vi "UHR-Fleezers Control (host) - 10.5.vi"() -> ()   [LabVIEW 2010] (continued)
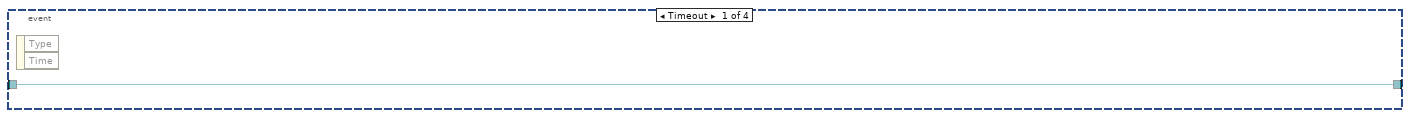
[diagram p2: hidden frame]
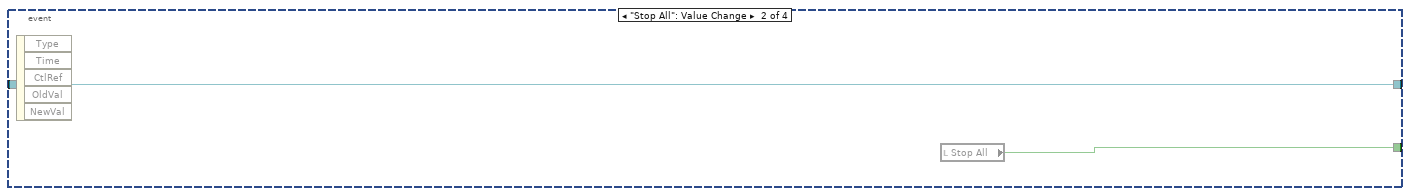
[diagram p3: hidden frame]
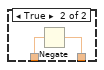
[diagram p4: hidden frame]
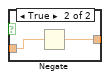
[diagram p5: hidden frame]
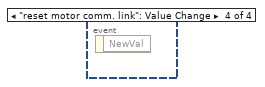
[diagram p6: hidden frame]
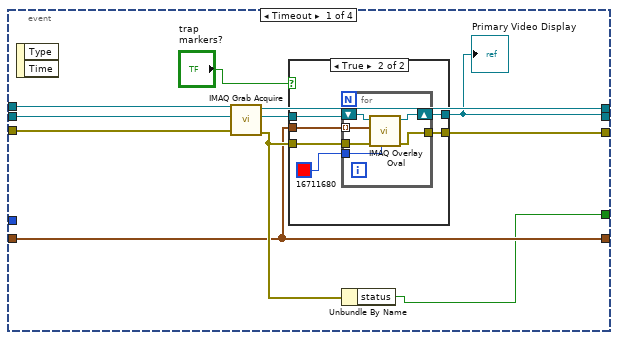
[diagram p8: hidden frame]
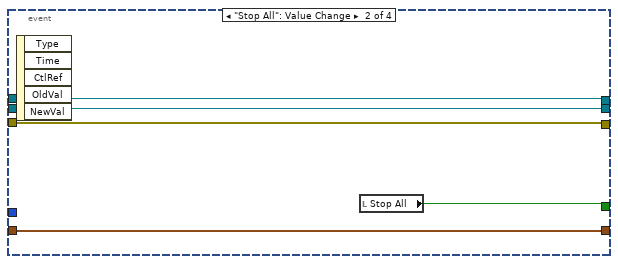
[diagram p10: hidden frame]
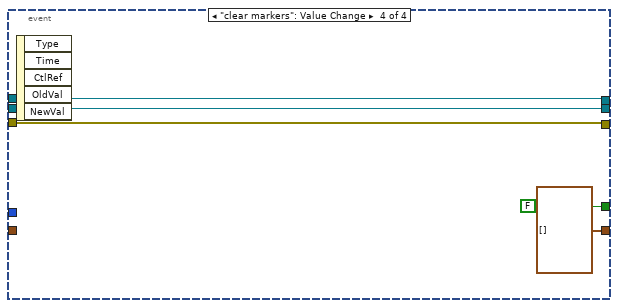
[diagram p12: hidden frame]
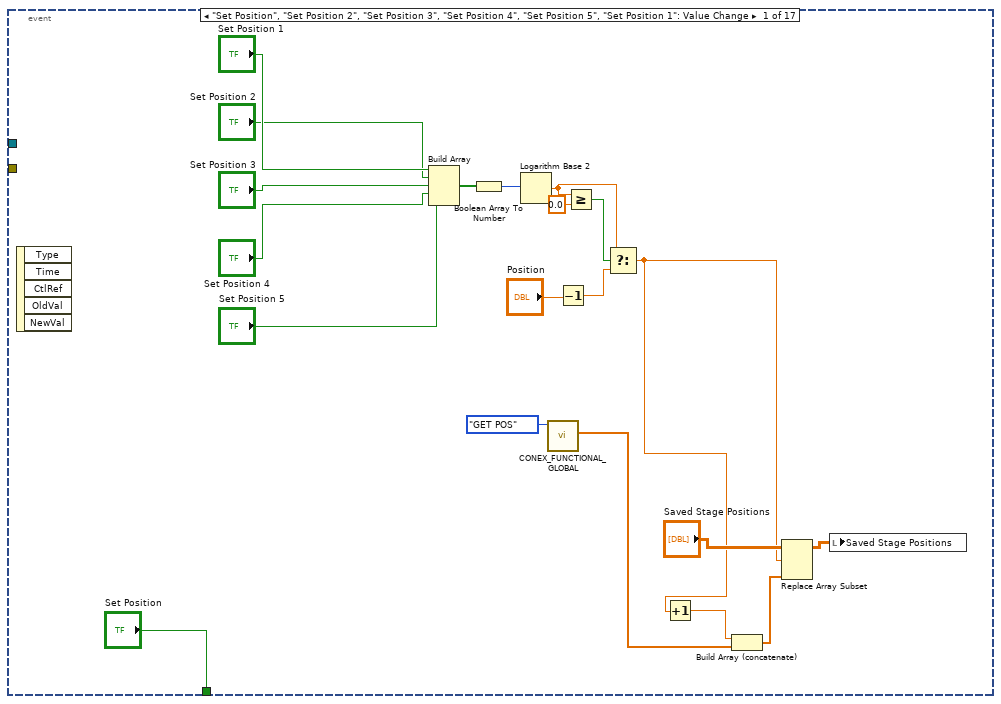
[diagram p13: hidden frame]
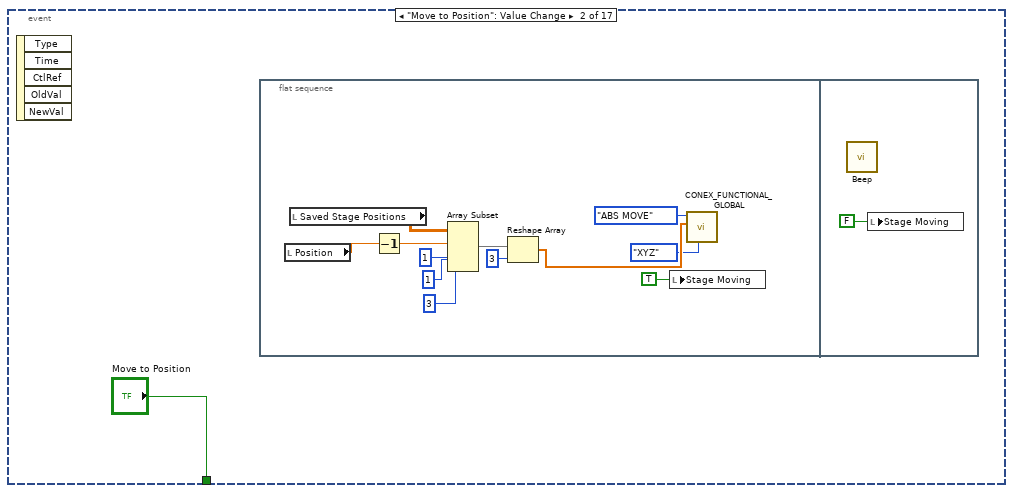
[diagram p14: hidden frame]
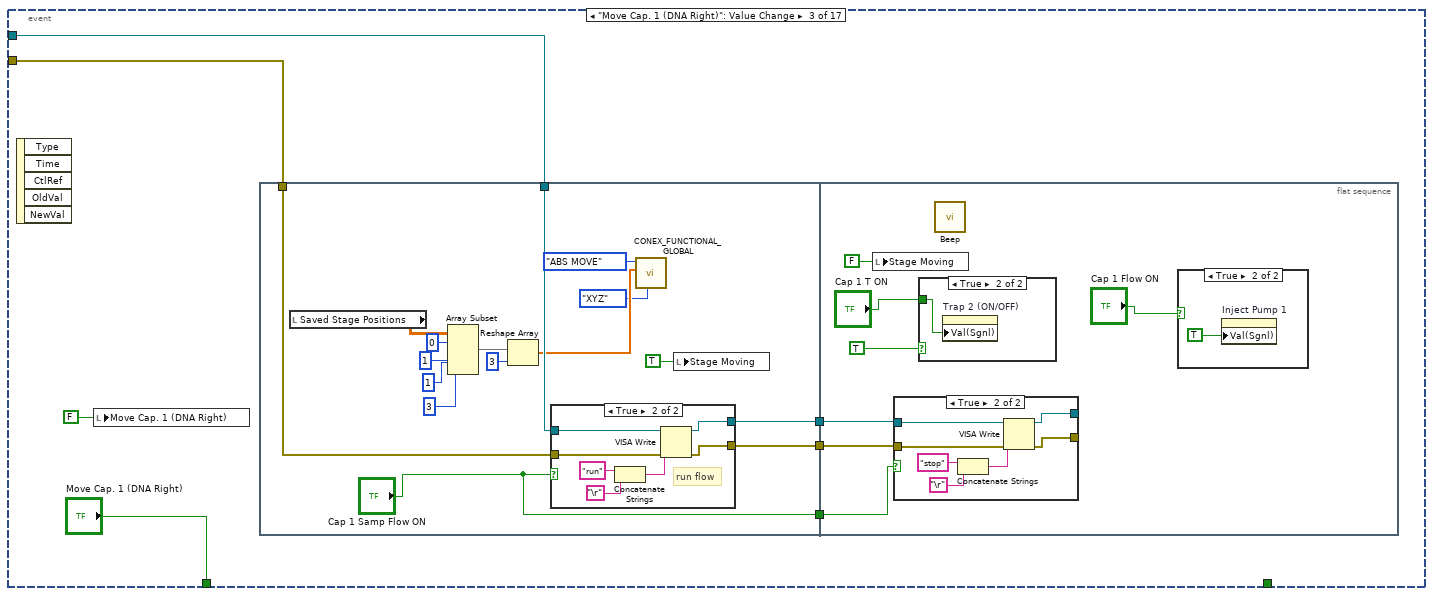
[diagram p15: hidden frame]
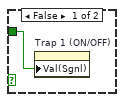
[diagram p19: hidden frame]
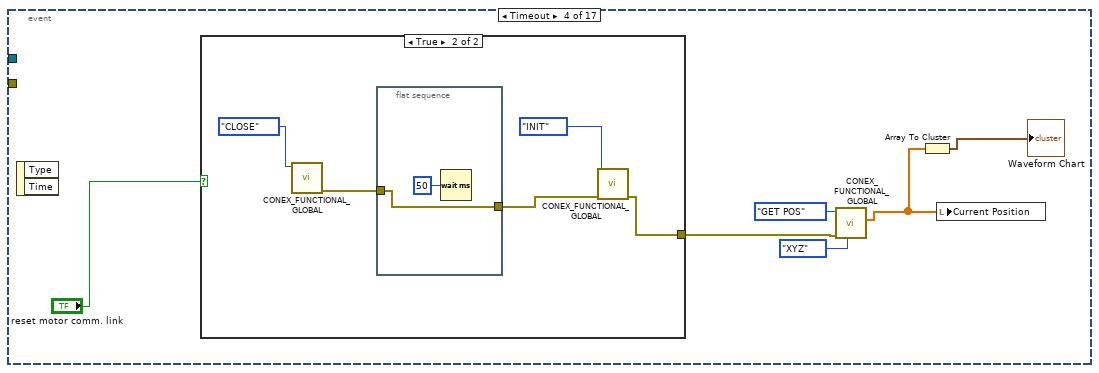
[diagram p20: hidden frame]
            n1941 = property on="Green laser mode" class="RadioBtnsControl (strict)"("Val(Sgnl)"=enum32{"Laser ON", "Laser OFF", "Interlace"}."Laser ON" ("Value (Signaling)")) -> ()  [unwired: 2 in, 2 out]
          }
          frame #3 {
            n1942 = Wait (ms)(milliseconds to wait=u32 500) -> ()  [unwired: 1 out]
          }
          frame #4 {
            n1943 = property on="Confocal Image" class="Bool (strict)"("Val(Sgnl)"=TRUE ("Value (Signaling)")) -> ()  [unwired: 2 in, 2 out]
          }
          frame #5 {
            n1944 = Wait (ms)(milliseconds to wait=u32 2000) -> ()  [unwired: 1 out]
          }
          frame #6 {
            n1945 = while {
              stop <- w8337 stop-if-true
              n1946 = local read "Saving..."() -> (w8338:bool)
              n1947 = Not(x=w8338) -> (.not. x?=w8337:bool)
            }
          }
          frame #7 {
            n1948 = property on="Flip Green Filter" class="Bool (strict)"("Val(Sgnl)"=TRUE ("Value (Signaling)")) -> ()  [unwired: 2 in, 2 out]
            n1949 = property on="Green Laser ON/Interlacing" class="Bool (strict)"("Val(Sgnl)"=w8342) -> ()  [unwired: 2 in, 2 out]
            n1950 = property on="Green laser mode" class="RadioBtnsControl (strict)"("Val(Sgnl)"=w8341) -> ()  [unwired: 2 in, 2 out]
          }
          frame #8 {
            n1951 = property on="Green FB On/Off" class="Bool (strict)"("Val(Sgnl)"=w8343) -> ()  [unwired: 2 in, 2 out]
          }
        }
      }
      event "Stop All": Value Change {
        n1952 = event-data() -> ()  [unwired: 1 in, 5 out]
        n1953 = local read "Stop All"() -> (w8344:bool)
      }
    }
    n1954 = node-c288() -> ()  [unwired: 1 in, 1 out]
  }
  n1955 = timed-loop "Mouse control: trap position (AOM deflection), set confocal spot from image" {
    tunnel: [w8346] -> w12
    tunnel: w9 -> [w8345]
    timing: w81 -> [_]
    timing-out: [_] -> w80
    stop <- w8346 stop-if-true
    n1956 = node-c288() -> ()  [unwired: 2 out]
    n1957 = event shown="[1] \"Pane\": Mouse Move" {
      selector: _ -> [_ _]
      dyn-events: _ -> [_ _]
      timeout: _ -> [_ _]
      tunnel: w8345 -> [w8349 _]
      event Mouse Down {
        n1958 = event-data() -> ("Time"=w8351:u32, "Coords"=w8350:T8, "Button"=w8352:u16)  [unwired: 6 out]
        n1959 = case shown="1" w8352 {
          tunnel: w8351 -> [_ _ w8455]
          tunnel: w8350 -> [_ w8389 w8453]
          tunnel: w8349 -> [_ _ w8451]
          frame 0, Default {
          }
          frame 1 {
            n1960 = property on="APD 2" class="ImageControl"() -> ("Displayed Image Position"=w8359:cluster{"Left":i32, "Top":i32})  [unwired: 2 in, 2 out]
            n1961 = property on="APD 1" class="ImageControl"() -> ("Displayed Image Position"=w8388:cluster{"Left":i32, "Top":i32})  [unwired: 2 in, 2 out]
            n1962 = property on="Detection Laser X" class="ImageControl"() -> ("Displayed Image Position"=w8385:cluster{"Left":i32, "Top":i32})  [unwired: 2 in, 2 out]
            n1963 = property on="Detection Laser Y" class="ImageControl"() -> ("Displayed Image Position"=w8384:cluster{"Left":i32, "Top":i32})  [unwired: 2 in, 2 out]
            n1964 = property on="APD 2" class="ImageControl"() -> ("Displayed Image Size"=w8358:cluster{"Width":u32, "Height":u32})  [unwired: 2 in, 2 out]
            n1965 = property on="APD 1" class="ImageControl"() -> ("Displayed Image Size"=w8386:cluster{"Width":u32, "Height":u32})  [unwired: 2 in, 2 out]
            n1966 = property on="Detection Laser X" class="ImageControl"() -> ("Displayed Image Size"=w8387:cluster{"Width":u32, "Height":u32})  [unwired: 2 in, 2 out]
            n1967 = property on="Detection Laser Y" class="ImageControl"() -> ("Displayed Image Size"=w8383:cluster{"Width":u32, "Height":u32})  [unwired: 2 in, 2 out]
            n1968 = Unbundle By Name(w8358) -> ("Width"=w8355:u32, "Height"=w8354:u32)
            n1969 = Unbundle By Name(w8359) -> ("Left"=w8357:i32, "Top"=w8356:i32)
            n1970 = Unbundle By Name(w8386) -> ("Width"=w8380:u32, "Height"=w8379:u32)
            n1971 = Unbundle By Name(w8387) -> ("Width"=w8376:u32, "Height"=w8375:u32)
            n1972 = Unbundle By Name(w8383) -> ("Width"=w8372:u32, "Height"=w8371:u32)
            n1973 = Unbundle By Name(w8388) -> ("Left"=w8382:i32, "Top"=w8381:i32)
            n1974 = Unbundle By Name(w8385) -> ("Left"=w8378:i32, "Top"=w8377:i32)
            n1975 = Unbundle By Name(w8384) -> ("Left"=w8374:i32, "Top"=w8373:i32)
            n1976 = Bundle("Left"=w8357, "Top"=w8356, "Width"=w8355, "Height"=w8354) -> (w8353:T50)  [unwired: 1 in]
            n1977 = Bundle("Left"=w8382, "Top"=w8381, "Width"=w8380, "Height"=w8379) -> (w8370:T50)  [unwired: 1 in]
            n1978 = Bundle("Left"=w8378, "Top"=w8377, "Width"=w8376, "Height"=w8375) -> (w8369:T50)  [unwired: 1 in]
            n1979 = Bundle("Left"=w8374, "Top"=w8373, "Width"=w8372, "Height"=w8371) -> (w8368:T50)  [unwired: 1 in]
            n1980 = Build Cluster Array(w8353, w8370, w8369, w8368) -> (w8367:T51)
            n1981 = for {
              tunnel: w8389 -> [w8400]
              tunnel: w8367 -> [w8401] mode=indexing
              shift-right: [w8398] -> w8365
              shift-left: TRUE -> [w8399]
              shift-right: [w8397] -> w8363
              shift-left: _ -> [w8393]
              shift-right: [w8396] -> w8362
              shift-left: _ -> [w8392]
              shift-right: [w8395] -> w8361
              shift-left: _ -> [w8391]
              shift-right: [w8394] -> w8360
              shift-left: _ -> [w8390]
              n1982 = case shown="True" w8399 {
                selector: w8399 -> [w8406 _]
                tunnel: w8401 -> [_ w8415]
                tunnel: w8400 -> [_ w8413]
                tunnel: [w8406 w8411] -> w8398
                tunnel: [w8405 w8410] -> w8397
                tunnel: [w8404 w8409] -> w8396
                tunnel: [w8403 w8408] -> w8395
                tunnel: [w8402 w8407] -> w8394
                tunnel: w8393 -> [w8405 _]
                tunnel: w8392 -> [w8404 _]
                tunnel: w8391 -> [w8403 _]
                tunnel: w8390 -> [w8402 _]
                frame False {
                }
                frame True {
                  n1983 = Unbundle(w8415) -> (w8414:T50)
                  n1984 = call "isclickinwindow.vi"("Image Param"=w8414, "Point32"=w8413) -> ("4 Y"=w8407:i32, "3 Height"=w8408:i32, "2 X"=w8409:i32, "1 Width"=w8410:i32, "In image?"=w8412:bool)  [unwired: 1 in]
                  n1985 = Not(x=w8412) -> (.not. x?=w8411:bool)
                }
              }
            }
            n1986 = Not(x=w8365) -> (.not. x?=w8364:bool)
            n1987 = case shown="True" w8364 {
              tunnel: w8362 -> [_ w8428]
              tunnel: w8360 -> [_ w8427]
              tunnel: w8363 -> [_ w8426]
              tunnel: w8361 -> [_ w8425]
              frame False {
              }
              frame True {
                w8421 = FALSE ("Get Point")
                n1988 = local read "Scan lines (y)"() -> (w8430:u64)
                n1989 = local read "Actual MCL Inc (V)"() -> (w8422:dbl)
                n1990 = local read "Scan steps (MCL)"() -> (w8429:u64)
                n1991 = Divide "Y Pix/step"(x=w8425, y=w8430) -> (x/y=w8437:dbl)
                n1992 = Divide "Y V/pix"(x=w8422, y=w8437) -> (x/y=w8436:dbl)
                n1993 = Divide "Y half step offset"(x=w8422, y=2.0) -> (x/y=w8438:dbl)
                n1994 = Divide "X pix/step"(x=w8426, y=w8429) -> (x/y=w8435:dbl)
                n1995 = Negate(x=w8438) -> (-x=w8439:dbl)
                n1996 = local read "Initial Y"() -> (w8445:dbl)
                n1997 = Multiply(x=w8427, y=w8436) -> (x*y=w8446:dbl)
                n1998 = Divide "X half step offset"(x=w8422, y=2.0) -> (x/y=w8432:dbl)
                n1999 = Divide "X V/pix"(x=w8422, y=w8435) -> (x/y=w8434:dbl)
                n2000 = Multiply(x=w8422, y=w8429) -> (x*y=w8441:dbl)
                n2001 = Compound Arithmetic op=ADD(w8439, w8446, w8445) -> (w8423:dbl)
                "Pointer Y (V)" <- w8423
                n2002 = Multiply(x=w8434, y=w8428) -> (x*y=w8443:dbl)
                n2003 = Negate(x=w8432) -> (-x=w8431:dbl)
                n2004 = local read "Initial X"() -> (w8444:dbl)
                n2005 = Negate(x=w8443) -> (-x=w8442:dbl)
                n2006 = Compound Arithmetic op=ADD(w8431, w8441, w8444, w8442) -> (w8424:dbl)
                "Pointer X (V)" <- w8424
                n2007 = Or(x="Set X Only", y="Set Confocal Spot (X-Y)") -> (x .or. y?=w8417:bool)
                n2008 = Or(x="Set Confocal Spot (X-Y)", y="Set Y Only") -> (x .or. y?=w8416:bool)
                n2009 = case shown="True" w8417 {
                  tunnel: w8424 -> [_ w8447]
                  frame False {
                  }
                  frame True {
                    n2010 = property on="AO2" class="Slide (strict)"("Val(Sgnl)"=w8447) -> ()  [unwired: 2 in, 2 out]
                  }
                }
                n2011 = case shown="True" w8416 {
                  tunnel: w8423 -> [_ w8448]
                  frame False {
                  }
                  frame True {
                    n2012 = property on="AO1" class="Slide (strict)"("Val(Sgnl)"=w8448) -> ()  [unwired: 2 in, 2 out]
                  }
                }
                n2013 = local write "Set Confocal Spot (X-Y)"(w8421) -> ()
                n2014 = local write "Set X Only"(w8421) -> ()
                n2015 = local write "Set Y Only"(w8421) -> ()
              }
            }
          }
          frame 3 {
            n2016 = local read "BD 2 Frequency 1 (MHz)"() -> (w8449:dbl)
            n2017 = local read "BD 1 Frequency 1 (MHz)"() -> (w8450:dbl)
            n2018 = local write "Manipulating Trap"(TRUE ("Manipulating Trap")) -> ()
            n2019 = local write "Coords"(T8 {"Horizontal"=0, "Vertical"=0} ("Coords")) -> ()
            n2020 = while {
              tunnel: w8455 -> [w8460]
              tunnel: w8453 -> [w8459]
              tunnel: w8451 -> [w8458]
              tunnel: w8450 -> [w8457]
              tunnel: w8449 -> [w8456]
              stop <- w8461 stop-if-true
              n2021 = event shown="[0] \"Pane\": Mouse Move" {
                selector: _ -> [_ _]
                dyn-events: _ -> [_ _]
                timeout: _ -> [_ _]
                tunnel: ["Force Manip Abort" w8525] -> w8461
                tunnel: w8460 -> [w8468 _]
                tunnel: w8459 -> [w8466 _]
                tunnel: w8458 -> [w8465 _]
                tunnel: w8457 -> [w8464 _]
                tunnel: w8456 -> [w8463 _]
                event Mouse Move {
                  n2022 = event-data() -> ("Time"=w8469:u32, "Coords"=w8470:T8)  [unwired: 3 out]
                  n2023 = Less?(x=w8469, y=w8468) -> (x < y?=w8467:bool)
                  n2024 = case "Makes sure old motion events prior to mouse click aren't used" shown="False" w8467 {
                    tunnel: w8470 -> [w8512 _]
                    tunnel: w8466 -> [w8513 _]
                    tunnel: w8465 -> [w8490 _]
                    tunnel: w8464 -> [w8486 _]
                    tunnel: w8463 -> [w8485 _]
                    frame False {
                      n2025 = Subtract(x=w8512, y=w8513) -> (x-y=w8511:T8)
                      "Coords" <- w8511
                      n2026 = local read "Y RF Frequency Limits (MHz)"() -> (w8471:T17)
                      n2027 = To Double Precision Float(number=w8511) -> (double precision float=w8510:cluster{"Horizontal":dbl, "Vertical":dbl})
                      n2028 = Multiply(x=cluster{"Horizontal":dbl, "Vertical":dbl} {"Horizontal"=-1.0, "Vertical"=1.0}, y="Manipulation Scaling") -> (x*y=w8506:cluster{"Horizontal":dbl, "Vertical":dbl})
                      n2029 = local read "X RF Frequency Limits (MHz)"() -> (w8472:T17)
                      n2030 = Multiply(x=w8510, y=w8506) -> (x*y=w8508:cluster{"Horizontal":dbl, "Vertical":dbl})
                      n2031 = Unbundle By Name(w8508) -> ("Horizontal"=w8503:dbl, "Vertical"=w8507:dbl)
                      n2032 = Unbundle By Name(w8471) -> ("Maximum"=w8474:dbl, "Minimum"=w8473:dbl)
                      n2033 = Boolean To (0,1)(Boolean="Manip. X?") -> (0, 1=w8501:i16)
                      n2034 = Boolean To (0,1)(Boolean="Manip. Y?") -> (0, 1=w8498:i16)
                      n2035 = local read "BD 1 Frequency 2 (MHz)"() -> (w8488:dbl)
                      n2036 = Multiply(x=w8507, y=w8498) -> (x*y=w8500:dbl)
                      n2037 = Multiply(x=w8501, y=w8503) -> (x*y=w8504:dbl)
                      n2038 = local read "BD 2 Frequency 2 (MHz)"() -> (w8487:dbl)
                      n2039 = Unbundle By Name(w8472) -> ("Maximum"=w8476:dbl, "Minimum"=w8475:dbl)
                      n2040 = Add(x=w8485, y=w8500) -> (x+y=w8478:dbl)
                      n2041 = Add(x=w8486, y=w8504) -> (x+y=w8480:dbl)
                      n2042 = In Range and Coerce(upper limit=w8476, x=w8480, lower limit=w8475) -> (coerced(x)=w8479:dbl)  [unwired: 1 out]
                      n2043 = In Range and Coerce(upper limit=w8474, x=w8478, lower limit=w8473) -> (coerced(x)=w8477:dbl)  [unwired: 1 out]
                      n2044 = Subtract(x=w8479, y=w8488) -> (x-y=w8497:dbl)
                      n2045 = Subtract(x=w8477, y=w8487) -> (x-y=w8496:dbl)
                      n2046 = Square(x=w8497) -> (x^2=w8495:dbl)
                      n2047 = Square(x=w8496) -> (x^2=w8494:dbl)
                      n2048 = Add(x=w8495, y=w8494) -> (x+y=w8493:dbl)
                      n2049 = Square Root(x=w8493) -> (sqrt(x)=w8489:dbl)
                      n2050 = In Range and Coerce(upper limit="Limit Max (MHz)", x=w8489, lower limit="Limit Min (MHz)") -> (In Range?=w8482:bool)  [unwired: 1 out]
                      n2051 = Not(x="Limits Enable") -> (.not. x?=w8481:bool)
                      n2052 = Or(x=w8482, y=w8481) -> (x .or. y?=w8483:bool)
                      n2053 = case shown="True" w8483 {
                        tunnel: w8490 -> [_ w8523]
                        tunnel: w8489 -> [_ w8514]
                        tunnel: w8479 -> [_ w8521]
                        tunnel: w8488 -> [_ w8520]
                        tunnel: w8477 -> [_ w8519]
                        tunnel: w8487 -> [_ w8518]
                        tunnel: w8472 -> [_ w8516]
                        tunnel: w8471 -> [_ w8515]
                        frame False {
                        }
                        frame True {
                          n2054 = local read "BD 1 Frequency 3 (MHz)"() -> (w8522:dbl)
                          n2055 = local read "BD 2 Frequency 3 (MHz)"() -> (w8517:dbl)
                          n2056 = local write "Trap Delta (MHz)"(w8514) -> ()
                          n2057 = property on="Initial delta (MHz)" class="DigNum (strict)"("Val(Sgnl)"=w8514) -> ()  [unwired: 2 in, 2 out]
                          n2058 = call "set RF board frequency - interlace.vi"("Board 2 Frequency Limits"=w8515, "Board 1 Frequency Limits"=w8516, "FPGA VI Reference In"=w8523, "Board 2 Frequency 3 (MHz)"=w8517, "Board 1 Frequency 3 (MHz)"=w8522, "Board 2 Frequency 2 (MHz)"=w8518, "Board 2 Frequency 1 (MHz)"=w8519, "Board 1 Frequency 2 (MHz)"=w8520, "Board 1 Frequency 1  (MHz)"=w8521) -> ()  [unwired: 1 in, 2 out]
                          n2059 = local write "BD 2 Frequency 1 (MHz)"(w8519) -> ()
                          n2060 = local write "BD 1 Frequency 1 (MHz)"(w8521) -> ()
                        }
                      }
                    }
                    frame True {
                    }
                  }
                }
                event Mouse Up {
                  n2061 = event-data() -> ("Button"=w8524:u16)  [unwired: 8 out]
                  n2062 = case shown="3" w8524 {
                    tunnel: [FALSE TRUE] -> w8525
                    frame 0, Default {
                    }
                    frame 3 {
                      n2063 = local write "Manipulating Trap"(FALSE ("Manipulating Trap")) -> ()
                    }
                  }
                }
              }
            }
          }
        }
      }
      event Mouse Move {
        n2064 = event-data() -> ()  [unwired: 6 out]
      }
    }
    n2065 = local read "Stop All"() -> (w8346:bool)
    n2066 = node-c288() -> ()  [unwired: 2 out]
  }
  n2067 = timed-loop "Oscillate AOD (debugging)" {
    tunnel: w9 -> [w8530]
    tunnel: [w8529] -> w14
    timing: w77 -> [_]
    timing-out: [_] -> w76
    stop <- w8529 stop-if-true
    n2068 = node-c288() -> ()  [unwired: 2 out]
    n2069 = event shown="[2] \"Stop All\": Value Change" {
      selector: _ -> [_ _ _]
      dyn-events: _ -> [_ _ _]
      timeout: _ -> [_ _ _]
      tunnel: w8530 -> [w8537 _ _]
      tunnel: [FALSE ("Stop All") _ w8806] -> w8529
      event "Oscillate Set 1", "Fish for Tether": Value Change {
        n2070 = event-data() -> ()  [unwired: 6 out]
        n2071 = local read "Oscillate Set 1"() -> (w8536:bool)
        n2072 = Or(x=w8536, y="Fish for Tether") -> (x .or. y?=w8534:bool)
        n2073 = case shown="True" w8534 {
          tunnel: w8537 -> [_ w8540]
          tunnel: "Fish for Tether" -> [_ w8539]
          frame False {
          }
          frame True {
            n2074 = case shown="False" w8539 {
              frame False {
              }
              frame True {
                n2075 = local write "Scan axis 2"(TRUE) -> ()
                n2076 = local write "Tether"(FALSE ("Tether")) -> ()
              }
            }
            n2077 = node-c288(i64 50 ("Period")) -> (w8542:T25)  [unwired: 3 out]
            n2078 = timed-loop "Oscillate AOD" {
              timing: w8542 -> [_]
              timing-out: [_] -> w8541
              tunnel: w8540 -> [w8552]
              tunnel: w8539 -> [w8551]
              i -> [w8554]
              stop <- w8550 stop-if-true
              n2079 = node-c288() -> (w8553:i64)  [unwired: 1 out]
              n2080 = flat-sequence {
                tunnel: w8554 -> [w8581]
                tunnel: w8553 -> [w8580]
                tunnel: w8552 -> [w8561]
                tunnel: w8551 -> [w8564]
                tunnel: [w8564] -> w8549
                tunnel: [w8563] -> w8548
                tunnel: [w8560] -> w8547
                tunnel: [w8557] -> w8545
                tunnel: w8549 -> [w8617]
                tunnel: w8548 -> [w8615]
                tunnel: w8547 -> [w8614]
                tunnel: [w8613] -> w8546
                tunnel: w8545 -> [w8612]
                tunnel: [w8681] -> w8550
                tunnel: w8546 -> [w8679]
                frame #0 {
                  n2081 = Divide(x=w8580, y=i64 1000) -> (x/y=w8575:dbl)
                  n2082 = Multiply(x=w8575, y=w8581) -> (x*y=w8577:dbl)
                  n2083 = Multiply(x="Osc. freq. (Hz)", y=6.283185307179586) -> (x*y=w8578:dbl)
                  n2084 = Multiply(x=w8578, y=w8577) -> (x*y=w8559:dbl)
                  n2085 = local read "BD 1 Frequency 2 (MHz)"() -> (w8562:dbl)
                  n2086 = local read "BD 1 Frequency 1 (MHz)"() -> (w8555:dbl)
                  n2087 = case shown="False" w8564 {
                    tunnel: w8559 -> [w8587 w8593]
                    tunnel: w8562 -> [_ w8604]
                    tunnel: [w8584 w8599] -> w8565
                    tunnel: [FALSE w8596] -> w8560
                    tunnel: [0.0 w8589] -> w8557
                    tunnel: w8555 -> [_ w8588]
                    frame False {
                      n2088 = Sine(x=w8587) -> (sin(x)=w8585:dbl)
                      n2089 = Multiply(x=w8585, y="Osc. amp. (MHz)") -> (x*y=w8584:dbl)
                    }
                    frame True {
                      n2090 = Cosine(x=w8593) -> (cos(x)=w8607:dbl)
                      n2091 = Subtract(x=w8604, y=w8588) -> (x-y=w8603:dbl)
                      n2092 = Decrement(x=w8607) -> (x-1=w8606:dbl)
                      n2093 = Subtract(x=w8603, y="Closest Delta (MHz)") -> (x-y=w8600:dbl)
                      n2094 = Divide(x=w8606, y=-2.0) -> (x/y=w8601:dbl)
                      n2095 = Multiply(x=w8601, y=w8600) -> (x*y=w8599:dbl)
                      n2096 = local read "Vec Mean of T1 T2"() -> (w8595:dbl[])
                      n2097 = Greater?(x=w8595, y="Stop F (pN)") -> (0:w8597:bool[])
                      n2098 = Or Array Elements(Boolean array=w8597) -> (logical OR=w8596:bool)
                      n2099 = Divide(x=w8593, y=6.283185307179586) -> (x/y=w8592:dbl)
                      n2100 = Round Toward +Infinity(x=w8592) -> (ceil(x): smallest int >= x=w8589:dbl)
                      "Attempts" <- w8589
                      n2101 = Greater?(x=w8589, y="Attempt Limit") -> (0:w8591:bool)
                      n2102 = case shown="True" w8591 {
                        frame False {
                        }
                        frame True {
                          n2103 = local write "Fish for Tether"(FALSE ("Fish for Tether")) -> ()
                          n2104 = call <vilib>:"Beep.vi"() -> ()  [unwired: 3 in, 9 out]
                          n2105 = local read "Messages"() -> (w8609:string)
                          n2106 = call "Update messages.vi"("Message to add"="Tether fishing timeout." ("Messages"), "Old message string"=w8609) -> ("New message string"=→"Messages":string)
                        }
                      }
                    }
                  }
                  n2107 = local read "BD 2 Frequency 1 (MHz)"() -> (w8566:dbl)
                  n2108 = Select(t=w8555, s="Scan axis 2", f=w8566) -> (s? t:f=w8569:dbl)
                  n2109 = Add(x=w8565, y=w8569) -> (x+y=w8563:dbl)
                  n2110 = Select(t=w8563, s="Scan axis 2", f=w8555) -> (s? t:f=w8556:dbl)
                  n2111 = Select(t=w8566, s="Scan axis 2", f=w8563) -> (s? t:f=w8571:dbl)
                  n2112 = local read "Y RF Frequency Limits (MHz)"() -> (w8567:T17)
                  n2113 = local read "X RF Frequency Limits (MHz)"() -> (w8568:T17)
                  n2114 = local read "BD 1 Frequency 3 (MHz)"() -> (w8574:dbl)
                  n2115 = local read "BD 2 Frequency 2 (MHz)"() -> (w8573:dbl)
                  n2116 = local read "BD 2 Frequency 3 (MHz)"() -> (w8572:dbl)
                  n2117 = call "set RF board frequency - interlace.vi"("Board 2 Frequency Limits"=w8567, "Board 1 Frequency Limits"=w8568, "FPGA VI Reference In"=w8561, "Board 2 Frequency 3 (MHz)"=w8572, "Board 1 Frequency 3 (MHz)"=w8574, "Board 2 Frequency 2 (MHz)"=w8573, "Board 2 Frequency 1 (MHz)"=w8571, "Board 1 Frequency 2 (MHz)"=w8562, "Board 1 Frequency 1  (MHz)"=w8556) -> ()  [unwired: 1 in, 2 out]
                }
                frame #1 {
                  n2118 = And(x=w8617, y=w8614) -> (x .and. y?=w8616:bool)
                  n2119 = case "Only if were fishing and now formed tether" shown="False" w8616 {
                    tunnel: w8615 -> [w8619 w8631]
                    tunnel: [w8618 w8630] -> w8613
                    tunnel: w8612 -> [_ w8626]
                    frame False {
                      n2120 = local read "Fish for Tether"() -> (w8618:bool)
                      n2121 = case shown="False" w8618 {
                        tunnel: w8619 -> [_ _]
                        frame False {
                        }
                        frame True {
                        }
                      }
                    }
                    frame True {
                      w8630 = FALSE ("Fish for Tether")
                      n2122 = call <vilib>:"Beep.vi"() -> ()  [unwired: 3 in, 9 out]
                      n2123 = Number To Decimal String(number=w8626, width (-)=i16 1) -> (decimal integer string=w8624:string)
                      n2124 = case shown="\"1\", Default" "Then..." {
                        selector: "Then..." -> [_ w8634]
                        tunnel: w8631 -> [w8633 _]
                        frame "1", Default {
                          n2125 = property on="BD 1 Frequency 1 (MHz)" class="DigNum (strict)"("Val(Sgnl)"=w8633) -> ()  [unwired: 2 in, 2 out]
                        }
                        frame "2", "3", "4", "5", "6" {
                          n2126 = flat-sequence {
                            tunnel: w8634 -> [w8636]
                            frame #0 {
                              n2127 = property on="Trap Delta (MHz)" class="DigNum (strict)"("Val(Sgnl)"="Move to Delta 1 (MHz)") -> ()  [unwired: 2 in, 2 out]
                            }
                            frame #1 {
                              n2128 = case shown="\"5\", \"6\"" w8636 {
                                selector: w8636 -> [w8639 w8649 _]
                                frame "3", "4" {
                                n2129 = flat-sequence {
                                tunnel: w8639 -> [w8640]
                                tunnel: [w8640] -> w8637
                                tunnel: [w8642] -> w8638
                                tunnel: w8637 -> [w8642]
                                tunnel: w8638 -> [w8646]
                                frame #0 {
                                n2130 = property on="Green Laser ON/Interlacing" class="Bool (strict)"("Val(Sgnl)"=TRUE ("Value (Signaling)")) -> ()  [unwired: 2 in, 2 out]
                                }
                                frame #1 {
                                n2131 = Multiply(x="Wait Before Save (s)", y=u32 1000 ("x")) -> (x*y=w8644:u32)
                                n2132 = Wait (ms)(milliseconds to wait=w8644) -> ()  [unwired: 1 out]
                                }
                                frame #2 {
                                n2133 = property on="Start Saving" class="Bool (strict)"("Value"=TRUE ("Start Saving")) -> ()  [unwired: 2 in, 2 out]
                                n2134 = case shown="\"4\"" w8646 {
                                frame Default {
                                }
                                frame "4" {
                                n2135 = property on="Fl. Triggered..." class="Bool (strict)"("Val(Sgnl)"=TRUE ("Value (Signaling)")) -> ()  [unwired: 2 in, 2 out]
                                }
                                }
                                }
                                }
                                }
                                frame "5", "6" {
                                n2136 = stacked-sequence {
                                tunnel: w8649 -> [_ _ _ _ _ _ _ _ w8666 _ _]
                                frame #0 {
                                n2137 = Replace Array Subset(array=u32[] [0] ("Index Values"), new element="Raster Set Upon Tether", index=0) -> (w8650:u32[])
                                n2138 = property on="Saved AOD Raster Scan Parameter Sets" class="Arr (strict)"("Index Values"=w8650) -> ()  [unwired: 2 in, 2 out]
                                }
                                frame #1 {
                                n2139 = Wait (ms)(milliseconds to wait=u32 500) -> ()  [unwired: 1 out]
                                }
                                frame #2 {
                                n2140 = property on="Load parameters" class="Bool (strict)"("Val(Sgnl)"=TRUE ("Value (Signaling)")) -> ()  [unwired: 2 in, 2 out]
                                }
                                frame #3 {
                                n2141 = Wait (ms)(milliseconds to wait=u32 500) -> ()  [unwired: 1 out]
                                }
                                frame #4 {
                                n2142 = property on="Trap Raster Scan" class="Bool (strict)"("Val(Sgnl)"=TRUE ("Value (Signaling)")) -> ()  [unwired: 2 in, 2 out]
                                }
                                frame #5 {
                                n2143 = Wait (ms)(milliseconds to wait=u32 2000) -> ()  [unwired: 1 out]
                                }
                                frame #6 {
                                n2144 = while {
                                stop <- w8661 stop-if-true
                                n2145 = local read "Raster Scanning..."() -> (w8660:bool)
                                n2146 = local read "Saving..."() -> (w8663:bool)
                                n2147 = Wait (ms)(milliseconds to wait=u32 100) -> ()  [unwired: 1 out]
                                n2148 = Not(x=w8663) -> (.not. x?=w8662:bool)
                                n2149 = Not(x=w8660) -> (.not. x?=w8659:bool)
                                n2150 = And(x=w8662, y=w8659) -> (x .and. y?=w8661:bool)
                                }
                                }
                                frame #7 {
                                n2151 = property on="Trap Delta (MHz)" class="DigNum (strict)"("Val(Sgnl)"="Move to Delta 2 (MHz)") -> ()  [unwired: 2 in, 2 out]
                                }
                                frame #8 {
                                n2152 = local read "Tether"() -> (w8667:bool)
                                n2153 = case shown="True" w8667 {
                                tunnel: w8666 -> [_ w8668]
                                frame False {
                                }
                                frame True {
                                n2154 = flat-sequence {
                                tunnel: w8668 -> [w8670]
                                frame #0 {
                                n2155 = Wait (ms)(milliseconds to wait=u32 500) -> ()  [unwired: 1 out]
                                }
                                frame #1 {
                                n2156 = case shown="\"6\"" w8670 {
                                frame Default {
                                }
                                frame "6" {
                                n2157 = property on="Green Laser ON/Interlacing" class="Bool (strict)"("Val(Sgnl)"=TRUE ("Green Laser ON/Interlacing")) -> ()  [unwired: 2 in, 2 out]
                                }
                                }
                                }
                                frame #2 {
                                n2158 = Wait (ms)(milliseconds to wait=u32 500) -> ()  [unwired: 1 out]
                                }
                                frame #3 {
                                n2159 = local write "Start Saving"("Save at end (5, 6)") -> ()
                                }
                                }
                                }
                                }
                                }
                                frame #9 {
                                n2160 = local read "Bead Sep. Int. Time (s)"() -> (w8676:dbl)
                                n2161 = Multiply(x=w8676, y=1000.0) -> (x*y=w8675:dbl)
                                n2162 = Wait (ms)(milliseconds to wait=w8675) -> ()  [unwired: 1 out]
                                }
                                frame #10 {
                                n2163 = property on="Rescale on Mean" class="Bool (strict)"("Val(Sgnl)"=TRUE ("Value (Signaling)")) -> ()  [unwired: 2 in, 2 out]
                                }
                                }
                                }
                                frame "2", Default {
                                }
                              }
                            }
                          }
                        }
                      }
                      n2164 = Concatenate Strings("Formed tether in ", w8624, " attempt(s)." ("string")) -> (w8621:string)
                      n2165 = local read "Messages"() -> (w8628:string)
                      n2166 = local write "Fish for Tether"(w8630) -> ()
                      n2167 = call "Update messages.vi"("Message to add"=w8621, "Old message string"=w8628) -> ("New message string"=w8627:string)
                      n2168 = local write "Messages"(w8627) -> ()
                      n2169 = Get Date/Time In Seconds() -> (seconds since 1Jan1904=→"Time tether formed":timestamp)
                      "Tether" <- "Tether Alarm?"
                    }
                  }
                }
                frame #2 {
                  n2170 = local read "Oscillate Set 1"() -> (w8680:bool)
                  n2171 = local read "Stop All"() -> (w8682:bool)
                  n2172 = Not Or(1:w8679, 2:w8680) -> (0:w8678:bool)
                  n2173 = Compound Arithmetic op=OR(w8682, w8678) -> (w8681:bool)
                }
              }
              n2174 = node-c288() -> ()  [unwired: 2 out]
            }
            n2175 = node-c288(w8541) -> ()  [unwired: 1 out]
          }
        }
      }
      event "Fl. Triggered...": Value Change {
        n2176 = event-data() -> ()  [unwired: 7 out]
        n2177 = case shown="True" "Fl. Triggered..." {
          frame False {
          }
          frame True {
            n2178 = node-c288() -> (w8694:T25)  [unwired: 4 out]
            n2179 = timed-loop {
              timing: w8694 -> [_]
              timing-out: [_] -> w8693
              tunnel: "Action" -> [w8698]
              shift-right: [w8695] -> _
              shift-left: u8 255 -> [w8697]
              stop <- w8699 stop-if-true
              n2180 = node-c288() -> ()  [unwired: 2 out]
              n2181 = flat-sequence {
                tunnel: w8698 -> [w8711]
                tunnel: w8697 -> [w8708]
                tunnel: [w8707] -> w8696
                tunnel: [w8797] -> w8699
                tunnel: w8696 -> [w8796]
                tunnel: [w8796] -> w8695
                frame #0 {
                  n2182 = local read "Delta Fl. 2"() -> (w8702:dbl)
                  n2183 = local read "Delta Fl. 1"() -> (w8703:dbl)
                  n2184 = Select(t=w8703, s="APD to Watch", f=w8702) -> (s? t:f=w8701:dbl)
                  n2185 = Multiply(x="Fl. Delta Thresh. (kHz)", y=1000.0) -> (x*y=w8710:dbl)
                  n2186 = Greater?(x=w8701, y=w8710) -> (0:w8705:bool)
                  n2187 = Or(x="Force Yank", y=w8705) -> (x .or. y?=w8706:bool)
                  n2188 = case shown="True" w8706 {
                    tunnel: w8711 -> [_ w8721]
                    tunnel: w8708 -> [w8713 w8717]
                    tunnel: [w8713 w8714] -> w8707
                    frame False {
                    }
                    frame True {
                      n2189 = flat-sequence {
                        tunnel: w8718 -> [w8727]
                        tunnel: [w8727] -> w8722
                        tunnel: w8721 -> [w8726]
                        tunnel: [w8726] -> w8720
                        tunnel: [w8725] -> w8719
                        tunnel: w8717 -> [w8724]
                        tunnel: [w8723] -> w8716
                        tunnel: w8722 -> [w8752]
                        tunnel: w8720 -> [w8751]
                        tunnel: w8719 -> [w8750]
                        tunnel: w8716 -> [w8749]
                        tunnel: [w8749] -> w8715
                        tunnel: w8715 -> [w8794]
                        tunnel: [w8794] -> w8714
                        frame #0 {
                          n2190 = call <vilib>:"Beep.vi"() -> ()  [unwired: 3 in, 9 out]
                          n2191 = local write "Waiting"(FALSE ("Waiting")) -> ()
                          n2192 = Increment(x=w8724) -> (x+1=w8723:u8)
                          n2193 = case shown="\"Yank\"" w8726 {
                            tunnel: w8723 -> [_ _ w8733]
                            frame "Image" {
                              n2194 = property on="Confocal Image" class="Bool (strict)"("Val(Sgnl)"=TRUE ("Value (Signaling)")) -> ()  [unwired: 2 in, 2 out]
                            }
                            frame "Alarm", Default {
                            }
                            frame "Yank" {
                              n2195 = flat-sequence {
                                tunnel: w8733 -> [w8736]
                                tunnel: [w8735] -> w8732
                                tunnel: ["N Array El"] -> w8731
                                tunnel: w8732 -> [w8746]
                                tunnel: w8731 -> [w8742]
                                frame #0 {
                                n2196 = Multiply(x="Yank Delay (s)", y=1000.0) -> (x*y=w8739:dbl)
                                n2197 = Quotient & Remainder(x=w8736, y="N Array El") -> (x-y*floor(x/y)=w8735:u8)  [unwired: 1 out]
                                n2198 = Wait (ms)(milliseconds to wait=w8739) -> ()  [unwired: 1 out]
                                }
                                frame #1 {
                                n2199 = Random Number (0-1)() -> (number: 0 to 1=w8743:dbl)
                                n2200 = Multiply(x=w8742, y=w8743) -> (x*y=w8741:dbl)
                                n2201 = Round Toward -Infinity(1:w8741) -> (0:w8740:dbl)
                                n2202 = Select(t=w8740, s="Random Choice", f=w8746) -> (s? t:f=w8744:dbl)
                                n2203 = Index Array(array="Yank to Delta Array (MHz)", index=w8744) -> (element=w8747:dbl)
                                n2204 = property on="Trap Delta (MHz)" class="DigNum (strict)"("Val(Sgnl)"=w8747) -> ()  [unwired: 2 in, 2 out]
                                }
                              }
                            }
                          }
                          n2205 = local read "Time (s)"() -> (w8725:dbl)
                          "Fl. High" <- TRUE ("Yanking")
                        }
                        frame #1 {
                          n2206 = node-c288() -> (w8754:T25)  [unwired: 4 out]
                          n2207 = timed-loop {
                            timing: w8754 -> [_]
                            timing-out: [_] -> w8753
                            tunnel: w8752 -> [w8770]
                            tunnel: w8751 -> [w8768]
                            tunnel: w8750 -> [w8767]
                            stop <- w8769 stop-if-true
                            n2208 = node-c288() -> ()  [unwired: 2 out]
                            n2209 = local read "Fl. Delta Thresh. (kHz)"() -> (w8762:dbl)
                            n2210 = local read "Fl. Triggered..."() -> (w8771:bool)
                            n2211 = local read "Delta Fl. 1"() -> (w8758:dbl)
                            n2212 = local read "Delta Fl. 2"() -> (w8756:dbl)
                            n2213 = local read "Stop All"() -> (w8765:bool)
                            n2214 = local read "APD to Watch"() -> (w8757:bool)
                            n2215 = Select(t=w8758, s=w8757, f=w8756) -> (s? t:f=w8755:dbl)
                            n2216 = Not(x=w8771) -> (.not. x?=w8766:bool)
                            n2217 = Multiply(x=w8762, y=1000.0) -> (x*y=w8761:dbl)
                            n2218 = Negate(x=w8761) -> (-x=w8760:dbl)
                            n2219 = Less?(x=w8755, y=w8760) -> (x < y?=w8764:bool)
                            n2220 = Compound Arithmetic op=OR(w8764, w8765, w8766, "Force Reset") -> (w8769:bool)
                            n2221 = case shown="True" w8769 {
                              tunnel: w8770 -> [_ w8782]
                              tunnel: w8768 -> [_ w8781]
                              tunnel: w8767 -> [_ w8779]
                              frame False {
                              }
                              frame True {
                                n2222 = case shown="\"Yank\"" w8781 {
                                tunnel: w8782 -> [_ w8783]
                                frame "Image", Default {
                                }
                                frame "Yank" {
                                n2223 = flat-sequence {
                                tunnel: [w8788] -> w8784
                                tunnel: w8783 -> [w8788]
                                tunnel: w8784 -> [w8789]
                                frame #0 {
                                n2224 = local read "Yank Delay (s)"() -> (w8787:dbl)
                                n2225 = Multiply(x=w8787, y=1000.0) -> (x*y=w8785:dbl)
                                n2226 = Wait (ms)(milliseconds to wait=w8785) -> ()  [unwired: 1 out]
                                }
                                frame #1 {
                                n2227 = property on="Trap Delta (MHz)" class="DigNum (strict)"("Val(Sgnl)"=w8789) -> ()  [unwired: 2 in, 2 out]
                                }
                                }
                                }
                                }
                                n2228 = local read "Time (s)"() -> (w8780:dbl)
                                n2229 = Subtract(x=w8780, y=w8779) -> (x-y=w8776:dbl)
                                "Duration (s)" <- w8776
                                n2230 = Number To Decimal String(number=w8776, width (-)=i16 0) -> (decimal integer string=w8774:string)
                                n2231 = Concatenate Strings(w8774, " s fluorescence event." ("string")) -> (w8772:string)
                                n2232 = local read "Messages"() -> (w8778:string)
                                n2233 = call "Update messages.vi"("Message to add"=w8772, "Old message string"=w8778) -> ("New message string"=w8777:string)
                                n2234 = call <vilib>:"Beep.vi"() -> ()  [unwired: 3 in, 9 out]
                                n2235 = local write "Messages"(w8777) -> ()
                              }
                            }
                            n2236 = node-c288() -> ()  [unwired: 2 out]
                          }
                          n2237 = node-c288(w8753) -> ()  [unwired: 1 out]
                        }
                        frame #2 {
                          n2238 = local write "Fl. High"(FALSE ("Yanking")) -> ()
                        }
                      }
                      n2239 = local read "Trap Delta (MHz)"() -> (w8718:dbl)
                    }
                  }
                }
                frame #1 {
                  n2240 = local read "Stop All"() -> (w8800:bool)
                  n2241 = local read "Fl. Triggered..."() -> (w8798:bool)
                  n2242 = Not(x=w8798) -> (.not. x?=w8799:bool)
                  n2243 = Or(x=w8799, y=w8800) -> (x .or. y?=w8797:bool)
                  n2244 = Not(x=w8797) -> (.not. x?=→"Waiting":bool)
                }
              }
              n2245 = node-c288() -> ()  [unwired: 2 out]
            }
            n2246 = node-c288(w8693) -> ()  [unwired: 1 out]
          }
        }
      }
      event "Stop All": Value Change {
        n2247 = event-data() -> ()  [unwired: 7 out]
        n2248 = local read "Stop All"() -> (w8806:bool)
      }
    }
    n2249 = node-c288() -> ()  [unwired: 2 out]
  }
  n2250 = node-c288(w31) -> ()  [unwired: 1 out]
  n2251 = call <vilib>:"IMAQ Stop.vi"("error in (no error)"=w18, "IMAQ Session In"=w20) -> ("error out"=w22:errorcluster, "IMAQ Session Out"=w21:refnum<k11>)  [unwired: 8 in]
  n2252 = call "IMAQ Dispose"("Image"=w19) -> ()  [unwired: 5 in, 1 out]
  n2253 = call <vilib>:"IMAQ Close.vi"("error in (no error)"=w22, "IMAQ Session In"=w21) -> ()  [unwired: 9 in, 1 out]
  n2254 = node-c288(w78) -> ()  [unwired: 1 out]
  n2255 = node-c288(w70) -> ()  [unwired: 1 out]
  n2256 = node-c288(w80) -> ()  [unwired: 1 out]
  n2257 = node-c288(w76) -> ()  [unwired: 1 out]
  n2258 = node-c288(w174) -> ()  [unwired: 1 out]
  n2259 = flat-sequence {
    tunnel: w11 -> [w8811]
    tunnel: [w8810] -> w17
    tunnel: [w8807] -> w16
    tunnel: w15 -> [_]
    tunnel: w14 -> [_]
    tunnel: w13 -> [_]
    tunnel: w12 -> [_]
    tunnel: w10 -> [w8808]
    tunnel: w17 -> [w8873]
    tunnel: w16 -> [w8872]
    frame #0 {
      w8809 = FALSE ("APD to FIFO")
      n2260 = xnode "Read/Write Control"("FPGA VI Reference In"=w8811, "error in"=w8808, "APD to FIFO"=w8809, "AI to FIFO"=w8809) -> ("FPGA VI Reference Out"=w8810:T20, "error out"=w8807:errorcluster)
    }
    frame #1 {
      n2261 = xnode "Invoke Method"("FPGA VI Reference In"=w8873, "error in"=w8872) -> ("FPGA VI Reference Out"=w8871:T20)  [unwired: 1 out]
      n2262 = xnode "Close FPGA VI Reference"("FPGA VI Reference In"=w8871) -> ()  [unwired: 1 in, 1 out]
    }
  }
